vi "HW_Loop_20181101.vi"(7 "ErrorLocation":string="FPGA", 8 "error in (no error)":errorcluster, 9 "10MHzPLL?":bool, 10 "FPGA.Target":T1=enum."4", 11 "Queue in":refnum<queue>) -> (0 "error out":errorcluster)   [LabVIEW 2018]
uses:
  Queue/HWQueueElements.ctl
  Controls/Enums/TargetNumber.ctl
  Controls/HWCluster.ctl
  Controls/Clusts/FPGA_Config_Clust.ctl
  Queue/DataQueueElements.ctl
  Controls/Enums/NoiseQueueElements.ctl
  Controls/Clusts/Config_Clust.ctl
  Controls/Clusts/UserConfig.ctl
  Controls/PathsCluster.ctl
  Controls/Clusts/FrontPanel_UserConfig.ctl
  Controls/Clusts/Inclinometer_User_Cfg.ctl
  Controls/Clusts/FP_UserTargetConfig.ctl
  Controls/Clusts/FreqShift.ctl
  Controls/Clusts/FPGA_Scale.ctl
  Controls/Enums/ScaleMeasure.ctl
  Controls/RadioButtons/FilterEnableRadio.ctl
  Controls/Enums/WatchdogTimer_Enum.ctl
  <vilib>/FPGAPlugInAG/PXIe-7976R/niLvFpga_Open_PXIe-7976R.vi
  <vilib>/rvi/interface/common/dynamic/niFpgaDynamicAddResources.vi
  <vilib>/FPGAPlugInAG/Dynamic/niLvFpga_Reset_Dynamic.vi
  <vilib>/FPGAPlugInAG/Dynamic/niLvFpga_Run_Dynamic.vi
  <vilib>/FPGAPlugInAG/Dynamic/niLvFpga_Close_Dynamic.vi
  <vilib>/rvi/interface/nirviOpenFPGA/nirviOpenFPGA.xnode
  FPGA Bitfiles/20210518_00_ATA_FPGA.lvbitx
  <vilib>/rvi/interface/nirviMethod/nirviMethod.xnode
  <vilib>/rvi/interface/nirviCloseFPGA/nirviCloseFPGA.xnode
  <vilib>/rvi/interface/nirviReadWriteControl/nirviReadWriteControl.xnode
  NiFpgaLv.dll
  <vilib>/Utility/error.llb/Error Cluster From Error Code.vi
  <vilib>/rvi/interface/Simulation/niFpgaSimulationCallBeginRW.vi
  <vilib>/rvi/errors/niLvFpgaAdjustHostInterfaceError.vi
panel:
  out "Synthesizer Locked":bool
  out "HWLoopCount":i32
  out "# elements in queue":i32
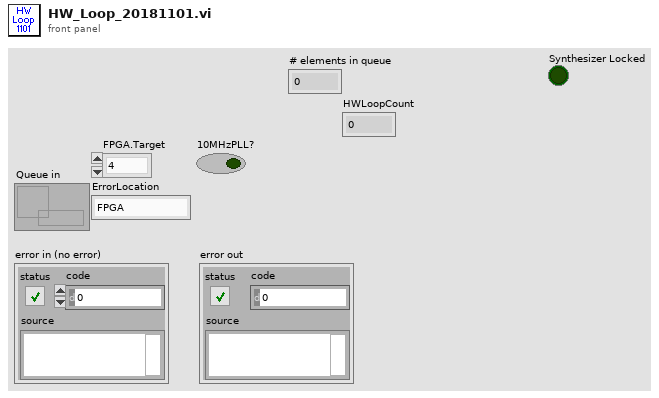
[diagram p1: front panel]
types:
  T1 = typedef "TargetNumber.ctl" = enum16{"1", "2", "3", "4"}
  T2 = typedef "HWCluster.ctl" = cluster{"FPGA":T3, "10MHzRef":bool, "FamInit":i32}
  T3 = typedef "FPGA_Config_Clust.ctl" = cluster{"Target":T1, "Channel":T1, "Ref1":refnum<k20>, "Ref2":refnum<k20>}
  T4 = typedef "HWQueueElements.ctl" = enum16{"HW_Init", "HW_UpdtCfg", "HW_Start", "HW_Pause", "HW_Run", "HW_Cls", "HW_Exit"}
  T5 = typedef "NoiseQueueElements.ctl" = enum16{"Noise_Startup", "Noise_Init", "Noise_Macro", "Noise_Config", "Noise_NewData", "Noise_Transform", "Noise_SumdTrace", "Noise_Send", "Noise_Probes", "Noise_Exit"}
  T6 = typedef "DataQueueElements.ctl" = enum16{"Data_Init", "Data_Config", "Data_AddData", "Data_FreqShift", "Data_FPGA_Write", "Data_Transform", "Data_Send", "Data_Exit"}
  T7 = enum8{"Internal Clock PLL Off", "Internal Clock PLL On (CLK_IN)", "External Clock (CLK_IN)", "Internal Clock PLL On (IoModSyncClk)"}
  T8 = typedef "Config_Clust.ctl" = cluster{"UsrCfg":T9, "FP_User":T11}
  T9 = typedef "UserConfig.ctl" = cluster{"Paths":T10, "SampleRate":dbl}
  T10 = typedef "PathsCluster.ctl" = cluster{"CfgFile":path, "LogFolder":path, "LogFile":path, "NAS path":path, "ThreshFile":path, "RedunFolder":path}
  T11 = typedef "FrontPanel_UserConfig.ctl" = cluster{"#NoiseSums":u32, "Max_df":u32, "AvgAvg":bool, "#Avg":u16, "AutoCenter":bool, "Inclin":T12, "1":T13, "2":T13, "3":T13, "4":T13, "Target to Probe":T1, "SNR_Thresh":dbl, "Paths":T10, "Connex_Location":string, "SimulateFPGA":bool, "Deadband":dbl}
  T12 = typedef "Inclinometer_User_Cfg.ctl" = cluster{"Vmin":dbl, "Vmax":dbl, "Angle_min":dbl, "Angle_max":dbl, "Offset":dbl, "Pos_Neg":bool}
  T13 = typedef "FP_UserTargetConfig.ctl" = cluster{"Cal_":T14, "Beac":T14, "Scale":T15, "Offset":fxp<+/-,16,16>, "Scale_Noise":fxp<+/-,30,30>, "Scale_Step1":fxp<+/-,17,17>, "Scale_In_RT":ext, "ScaleMeas":fxp<+/-,16,1>, "FreqsToRemove":i32[], "Width":i32[], "ScaleMeasEnum":T16, "FilterEnab":T17}
  T14 = typedef "FreqShift.ctl" = cluster{"Fine":dbl, "Coarse_":dbl}
  T15 = typedef "FPGA_Scale.ctl" = cluster{"Step4":fxp<+/-,23,23>, "Step5":fxp<+/-,23,23>, "Step6":fxp<+/-,23,23>, "Step7":fxp<+/-,23,23>}
  T16 = typedef "ScaleMeasure.ctl" = enum16{"1", "10", "50", "42"}
  T17 = typedef "FilterEnableRadio.ctl" = enum32{"None", "Step 1", "Frequency Shift", "Step 4", "Step 5", "Step 6", "Step 7"}
  T18 = typedef "WatchdogTimer_Enum.ctl" = enum16{"ResetAll", "CheckAll", "HW1", "HW2", "Tones", "FP", "Noise", "Log", "TCP", "AI", "TC", "ADAM", "Disdrom", "TE", "Weather"}
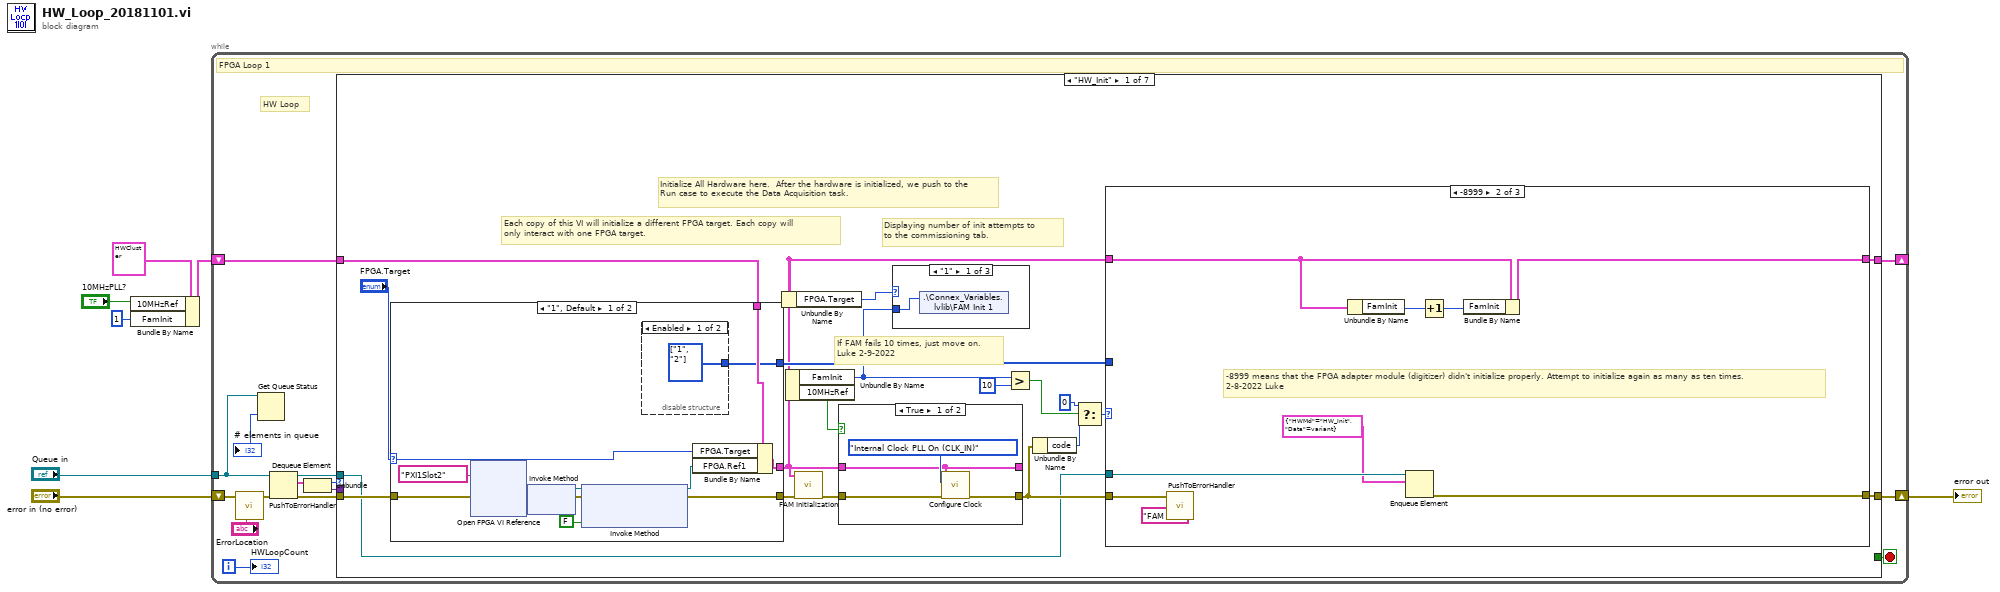
[diagram p0: block diagram]
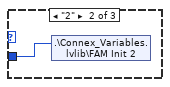
[diagram p2: hidden frame]
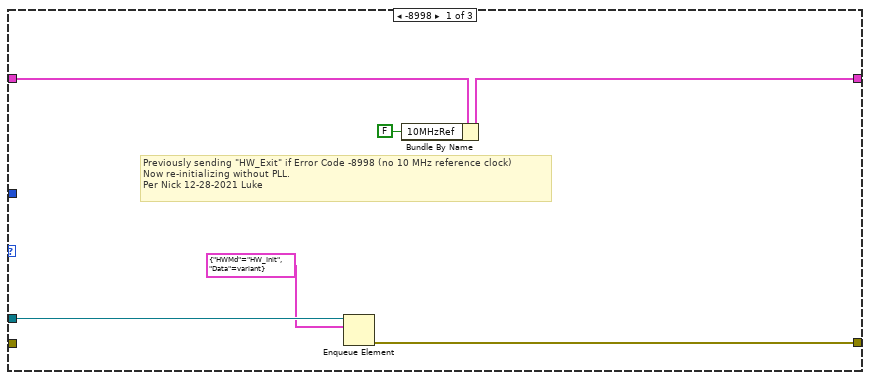
[diagram p4: hidden frame]
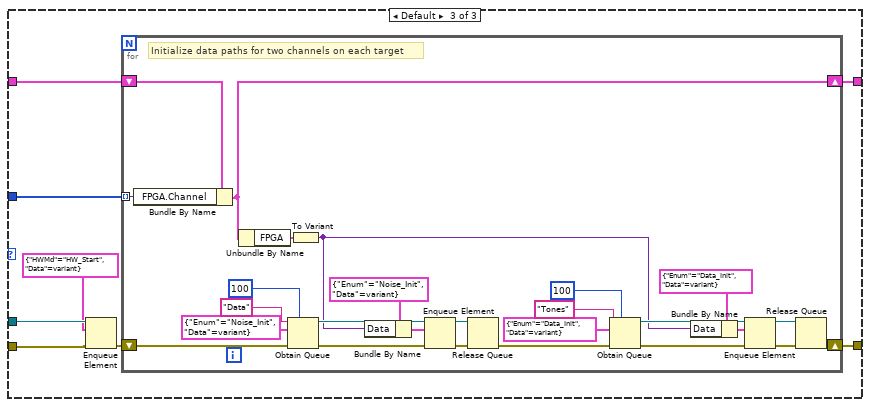
[diagram p5: hidden frame]
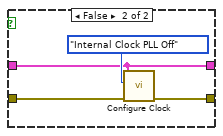
[diagram p6: hidden frame]
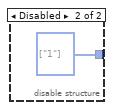
[diagram p7: hidden frame]
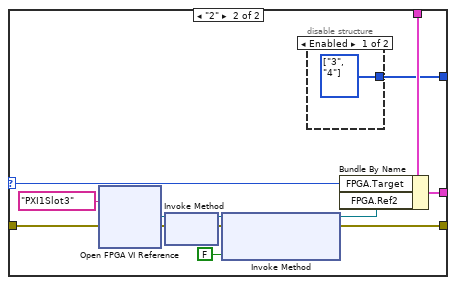
[diagram p8: hidden frame]
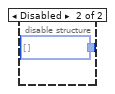
[diagram p9: hidden frame]
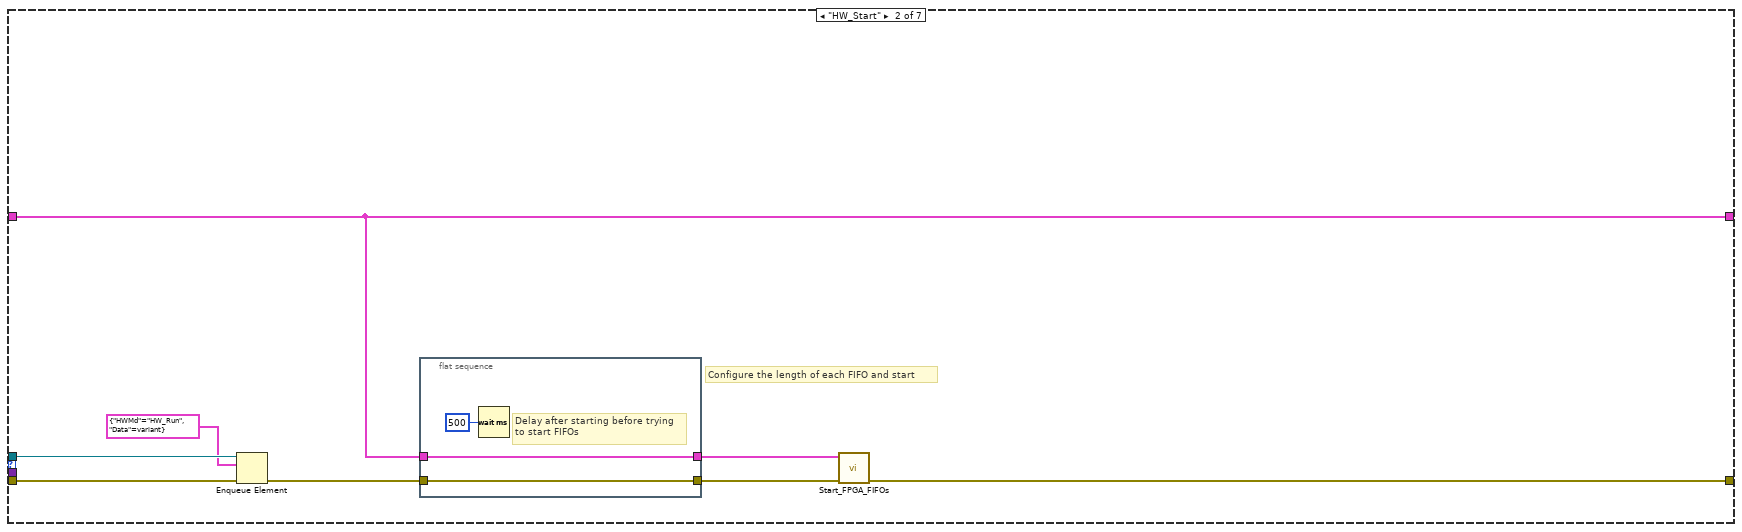
[diagram p10: hidden frame]
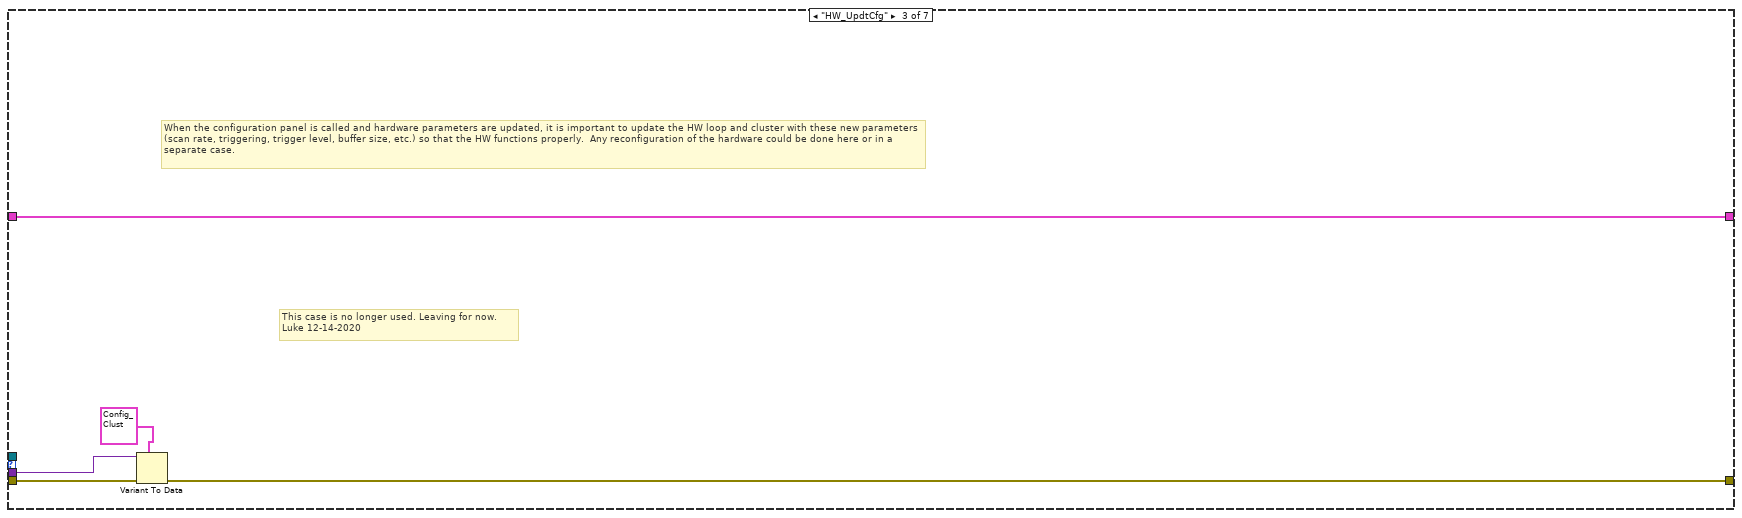
[diagram p11: hidden frame]
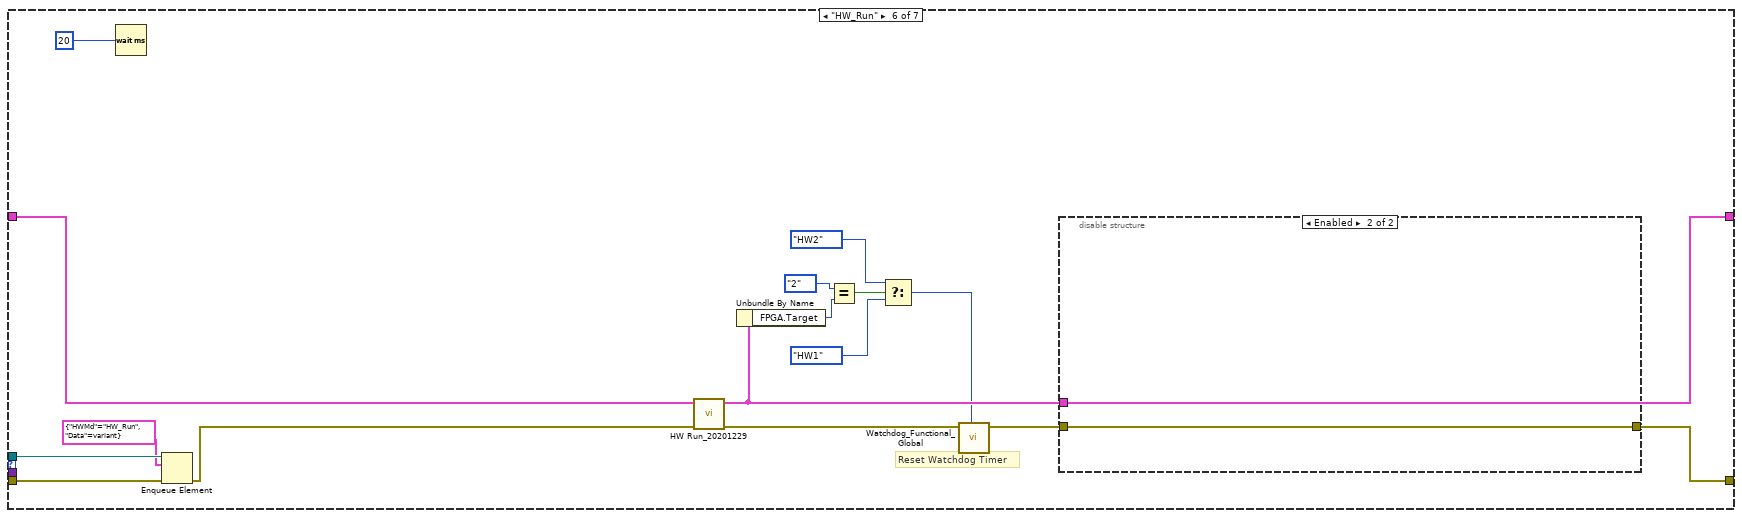
[diagram p14: hidden frame]
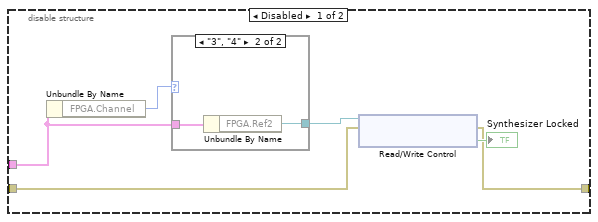
[diagram p15: hidden frame]
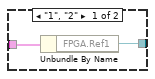
[diagram p16: hidden frame]
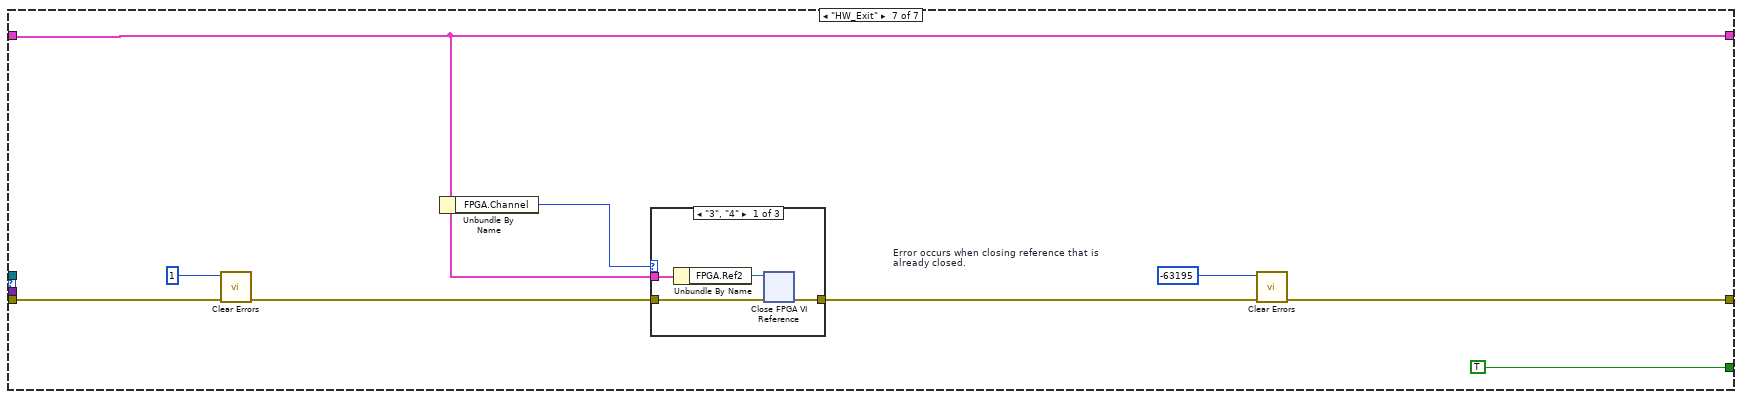
[diagram p17: hidden frame]
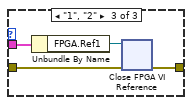
[diagram p19: hidden frame]
diagram:
  n1 = Bundle By Name(cluster=T2 {"FPGA"={"Target"=enum."4", "Channel"=enum."4", "Ref1"=refnum, "Ref2"=refnum}, "10MHzRef"=FALSE, "FamInit"=0} ("ClusterOut"), "10MHzRef"="10MHzPLL?", "FamInit"=1) -> (w3:T2)
  n2 = while {
    shift-right: [w12] -> w6
    shift-left: "error in (no error)" -> [w14]
    shift-right: [w22] -> _
    shift-left: w3 -> [w19]
    tunnel: "Queue in" -> [w10]
    i -> [w8]
    stop <- w15 stop-if-true
    # "HW Loop"
    # "FPGA Loop 1"
    n3 = call "PushToErrorHandler.vi"("ErrorIn"=w14, "ErrorLocation"="ErrorLocation") -> ("ErrorOut"=w13:errorcluster)  [unwired: 5 in]
    n4 = Get Queue Status(queue=w10) -> (# elements in queue=→"# elements in queue":i32)  [unwired: 2 in, 7 out]
    n5 = Dequeue Element(queue=w10, error in (no error)=w13) -> (queue out=w17:refnum<queue>, element=w21:cluster{"HWMd":T4, "Data":variant}, error out=w18:errorcluster)  [unwired: 2 out]
    n6 = Unbundle(w21) -> ("HWMd"=w20:T4, "Data"=w16:variant)
    n7 = case shown="\"HW_Init\"" w20 {
      tunnel: [w37 w138 w145 w148 w150 w160 w181] -> w12
      tunnel: [w36 w136 w142 w147 w149 w157 w179] -> w22
      tunnel: w19 -> [w39 w136 w142 w147 w149 w162 w179]
      tunnel: w18 -> [w41 w133 w146 w148 w150 w166 w178]
      tunnel: w17 -> [w31 w132 _ _ _ w165 _]
      tunnel: w16 -> [_ _ w144 _ _ _ _]
      tunnel: [_ _ _ _ _ _ TRUE ("Exit?")] -> w15
      frame "HW_Init" {
        # "Displaying number of init attempts to\nto the commissioning tab."
        # "If FAM fails 10 times, just move on.\nLuke 2-9-2022"
        # "Each copy of this VI will initialize a different FPGA target. Each copy will\nonly interact with one FPGA target."
        # "Initialize All Hardware here.  After the hardware is initialized, we push to the Run case to execute the Data Acquisition task."
        n8 = case shown="\"1\", Default" "FPGA.Target" {
          selector: "FPGA.Target" -> [w108 w123]
          tunnel: w41 -> [w113 w128]
          tunnel: [w103 w117] -> w38
          tunnel: w39 -> [w111 w127]
          tunnel: [w110 w126] -> w25
          tunnel: [w109 w124] -> w35
          frame "1", Default {
            n9 = xnode ("Open FPGA VI Reference")("error in"=w113, "resource name"=tag "PXI1Slot2") -> ("FPGA VI Reference Out"=w106:refnum<k20>, "error out"=w107:errorcluster)
            n10 = xnode "Invoke Method"("FPGA VI Reference In"=w106, "error in"=w107) -> ("FPGA VI Reference Out"=w104:refnum<k20>, "error out"=w105:errorcluster)
            n11 = xnode "Invoke Method"("FPGA VI Reference In"=w104, "error in"=w105, "Wait Until Done (F)"=FALSE) -> ("FPGA VI Reference Out"=w101:refnum<k20>, "error out"=w103:errorcluster)
            n12 = disable-structure shown="Enabled" {
              disable-tunnel: [w114 w115] -> w109
              frame Enabled {
                w114 = T1[] [enum."1", enum."2"] items=["1", "2", "3", "4"]
              }
              frame Disabled {
                w115 = T1[] [enum."1"] items=["1", "2", "3", "4"]
              }
            }
            n13 = Bundle By Name(cluster=w111, "FPGA.Target"=w108, "FPGA.Ref1"=w101) -> (w110:T2)
          }
          frame "2" {
            n14 = xnode ("Open FPGA VI Reference")("error in"=w128, "resource name"=tag "PXI1Slot3") -> ("FPGA VI Reference Out"=w121:refnum<k20>, "error out"=w122:errorcluster)
            n15 = xnode "Invoke Method"("FPGA VI Reference In"=w121, "error in"=w122) -> ("FPGA VI Reference Out"=w119:refnum<k20>, "error out"=w120:errorcluster)
            n16 = xnode "Invoke Method"("FPGA VI Reference In"=w119, "error in"=w120, "Wait Until Done (F)"=FALSE) -> ("FPGA VI Reference Out"=w118:refnum<k20>, "error out"=w117:errorcluster)
            n17 = disable-structure shown="Enabled" {
              disable-tunnel: [w129 w130] -> w124
              frame Enabled {
                w129 = T1[] [enum."3", enum."4"] items=["1", "2", "3", "4"]
              }
              frame Disabled {
                w130 = T1[] [] items=["1", "2", "3", "4"]
              }
            }
            n18 = Bundle By Name(cluster=w127, "FPGA.Target"=w123, "FPGA.Ref2"=w118) -> (w126:T2)
          }
        }
        n19 = Unbundle By Name(w25) -> ("FPGA.Target"=w24:T1)
        n20 = Unbundle By Name(w25) -> ("FamInit"=w23:i32, "10MHzRef"=w33:bool)
        n21 = call "FAM Initialization.vi"("error in (no error)"=w38, "Cluster"=w25) -> ("error out"=w34:errorcluster)  [unwired: 8 in, 1 out]
        n22 = case shown="True" w33 {
          tunnel: w34 -> [w94 w98]
          tunnel: [w95 w99] -> w32
          tunnel: w25 -> [w93 w97]
          tunnel: [w93 w97] -> _
          frame True {
            n23 = call "Configure Clock.vi"("error in"=w94, "Clock Source"=T7."Internal Clock PLL On (CLK_IN)", "Cluster"=w93) -> ("error out"=w95:errorcluster)  [unwired: 7 in, 1 out]
          }
          frame False {
            n24 = call "Configure Clock.vi"("error in"=w98, "Clock Source"=T7."Internal Clock PLL Off", "Cluster"=w97) -> ("error out"=w99:errorcluster)  [unwired: 7 in, 1 out]
          }
        }
        n25 = case shown="\"1\"" w24 {
          tunnel: w23 -> [w42 w43 _]
          frame "1" {
            n26 = shared-variable ".\\Connex_Variables.lvlib\\FAM Init 1"(w42) -> ()  [unwired: 1 in, 1 out]
          }
          frame "2" {
            n27 = shared-variable ".\\Connex_Variables.lvlib\\FAM Init 2"(w43) -> ()  [unwired: 1 in, 1 out]
          }
          frame Default {
          }
        }
        n28 = Greater?(x=w23, y=10) -> (0:w29:bool)
        n29 = Unbundle By Name(w32) -> ("code"=w28:i32)
        n30 = Select(t=0, s=w29, f=w28) -> (s? t:f=w27:i32)
        n31 = case shown="-8999" w27 {
          tunnel: [w48 w57 w66] -> w37
          tunnel: [w46 w56 w65] -> w36
          tunnel: w35 -> [_ _ w64]
          tunnel: w32 -> [_ w51 w61]
          tunnel: w25 -> [w47 w54 w63]
          tunnel: w31 -> [w49 w58 w60]
          frame -8998 {
            # "Previously sending \"HW_Exit\" if Error Code -8998 (no 10 MHz reference clock)\nNow re-initializing without PLL. \nPer Nick 12-28-2021 Luke"
            n32 = Enqueue Element(queue=w49, element=cluster{"HWMd":T4, "Data":variant} {"HWMd"=enum."HW_Init", "Data"=variant}) -> (error out=w48:errorcluster)  [unwired: 1 in, 3 out]
            n33 = Bundle By Name(cluster=w47, "10MHzRef"=FALSE) -> (w46:T2)
          }
          frame -8999 {
            # "-8999 means that the FPGA adapter module (digitizer) didn't initialize properly. Attempt to initialize again as many as ten times.\n2-8-2022 Luke"
            n34 = call "PushToErrorHandler.vi"("ErrorIn"=w51, "ErrorLocation"="FAM Init") -> ()  [unwired: 5 in, 1 out]
            n35 = Unbundle By Name(w54) -> ("FamInit"=w53:i32)
            n36 = Enqueue Element(queue=w58, element=cluster{"HWMd":T4, "Data":variant} {"HWMd"=enum."HW_Init", "Data"=variant}) -> (error out=w57:errorcluster)  [unwired: 1 in, 3 out]
            n37 = Increment(x=w53) -> (x+1=w52:i32)
            n38 = Bundle By Name(cluster=w54, "FamInit"=w52) -> (w56:T2)
          }
          frame Default {
            n39 = Enqueue Element(queue=w60, element=cluster{"HWMd":T4, "Data":variant} {"HWMd"=enum."HW_Start", "Data"=variant}, error in (no error)=w61) -> (error out=w62:errorcluster)  [unwired: 3 out]
            n40 = for {
              shift-right: [w71] -> w66
              shift-left: w62 -> [w76]
              shift-right: [w68] -> w65
              shift-left: w63 -> [w69]
              tunnel: w64 -> [w67] mode=indexing
              # "Initialize data paths for two channels on each target"
              n41 = Bundle By Name(cluster=w69, "FPGA.Channel"=w67) -> (w68:T2)
              n42 = Unbundle By Name(w68) -> ("FPGA"=w81:T3)
              n43 = Obtain Queue(max queue size (-1, unlimited)=100, name (unnamed)="Data", element data type=cluster{"Enum":T5, "Data":variant} {"Enum"=enum."Noise_Init", "Data"=variant}, error in (no error)=w76) -> (queue out=w80:refnum<queue>, error out=w82:errorcluster)  [unwired: 1 in, 1 out]
              n44 = To Variant(anything=w81) -> (Variant=w77:variant)
              n45 = Bundle By Name(cluster=cluster{"Enum":T5, "Data":variant} {"Enum"=enum."Noise_Init", "Data"=variant} ("element"), "Data"=w77) -> (w78:cluster{"Enum":T5, "Data":variant})
              n46 = Enqueue Element(queue=w80, element=w78, error in (no error)=w82) -> (queue out=w73:refnum<queue>, error out=w75:errorcluster)  [unwired: 2 out]
              n47 = Release Queue(queue=w73, error in (no error)=w75) -> (error out=w74:errorcluster)  [unwired: 1 in, 2 out]
              n48 = Obtain Queue(max queue size (-1, unlimited)=100, name (unnamed)="Tones", element data type=cluster{"Enum":T6, "Data":variant} {"Enum"=enum."Data_Init", "Data"=variant}, error in (no error)=w74) -> (queue out=w86:refnum<queue>, error out=w87:errorcluster)  [unwired: 1 in, 1 out]
              n49 = Bundle By Name(cluster=cluster{"Enum":T6, "Data":variant} {"Enum"=enum."Data_Init", "Data"=variant} ("element"), "Data"=w77) -> (w91:cluster{"Enum":T6, "Data":variant})
              n50 = Enqueue Element(queue=w86, element=w91, error in (no error)=w87) -> (queue out=w70:refnum<queue>, error out=w72:errorcluster)  [unwired: 2 out]
              n51 = Release Queue(queue=w70, error in (no error)=w72) -> (error out=w71:errorcluster)  [unwired: 1 in, 2 out]
            }
          }
        }
      }
      frame "HW_Start" {
        # "Configure the length of each FIFO and start"
        n52 = Enqueue Element(queue=w132, element=cluster{"HWMd":T4, "Data":variant} {"HWMd"=enum."HW_Run", "Data"=variant}, error in (no error)=w133) -> (error out=w134:errorcluster)  [unwired: 1 in, 2 out]
        n53 = flat-sequence {
          tunnel: w134 -> [w140]
          tunnel: [w140] -> w137
          tunnel: w136 -> [w139]
          tunnel: [w139] -> w135
          frame #0 {
            # "Delay after starting before trying\nto start FIFOs"
            n54 = Wait (ms)(milliseconds to wait=u32 500) -> ()  [unwired: 1 out]
          }
        }
        n55 = call "Start_FPGA_FIFOs.vi"("error in (no error)"=w137, "ClusterOut"=w135) -> ("error out"=w138:errorcluster)  [unwired: 9 in]
      }
      frame "HW_UpdtCfg" {
        # "This case is no longer used. Leaving for now.\nLuke 12-14-2020"
        # "When the configuration panel is called and hardware parameters are updated, it is important to update the HW loop and cluster with these new parameters (scan rate, triggering, trigger level, buffer size, etc.) so that the HW functions properly.  Any reconfiguration of the hardware could be done here or in a separate case."
        n56 = Variant To Data(error in=w146, type=T8 {"UsrCfg"={"Paths"={"CfgFile"=path "", "LogFolder"=path "", "LogFile"=path "", "NAS path"=path "", "ThreshFile"=path "", "RedunFolder"=path ""}, "SampleRate"=12500.0}, "FP_User"={"#NoiseSums"=1, "Max_df"=1, "AvgAvg"=FALSE, "#Avg"=1, "AutoCenter"=FALSE, "Inclin"={"Vmin"=0.0, "Vmax"=0.0, "Angle_min"=0.0, "Angle_max"=0.0, "Offset"=0.0, "Pos_Neg"=FALSE}, "1"={"Cal_"={"Fine"=0.000213623046875, "Coarse_"=4194303.0}, "Beac"={"Fine"=4194303.0, "Coarse_"=1.0}, "Scale"={"Step4"=10000.0, "Step5"=4194303.0, "Step6"=1.0, "Step7"=10000.0}, "Offset"=0.0, "Scale_Noise"=4194303.0, "Scale_Step1"=65535.0, "Scale_In_RT"=1.0, "ScaleMeas"=0.999969482421875, "FreqsToRemove"=[0, 1633], "Width"=[0, 1633], "ScaleMeasEnum"=enum."50", "FilterEnab"=enum."Step 1"}, "2"={"Cal_"={"Fine"=0.000213623046875, "Coarse_"=4194303.0}, "Beac"={"Fine"=0.000213623046875, "Coarse_"=4194303.0}, "Scale"={"Step4"=0.0, "Step5"=4194303.0, "Step6"=1.0, "Step7"=10000.0}, "Offset"=0.0, "Scale_Noise"=4194303.0, "Scale_Step1"=65535.0, "Scale_In_RT"=1.0, "ScaleMeas"=0.999969482421875, "FreqsToRemove"=[0, 1633], "Width"=[0, 1633], "ScaleMeasEnum"=enum."50", "FilterEnab"=enum."Step 1"}, "3"={"Cal_"={"Fine"=0.000213623046875, "Coarse_"=4194303.0}, "Beac"={"Fine"=0.000213623046875, "Coarse_"=4194303.0}, "Scale"={"Step4"=0.0, "Step5"=4194303.0, "Step6"=1.0, "Step7"=10000.0}, "Offset"=0.0, "Scale_Noise"=4194303.0, "Scale_Step1"=65535.0, "Scale_In_RT"=1.0, "ScaleMeas"=0.999969482421875, "FreqsToRemove"=[0, 1633], "Width"=[0, 1633], "ScaleMeasEnum"=enum."50", "FilterEnab"=enum."Step 1"}, "4"={"Cal_"={"Fine"=0.000213623046875, "Coarse_"=4194303.0}, "Beac"={"Fine"=0.000213623046875, "Coarse_"=4194303.0}, "Scale"={"Step4"=0.0, "Step5"=4194303.0, "Step6"=1.0, "Step7"=10000.0}, "Offset"=0.0, "Scale_Noise"=4194303.0, "Scale_Step1"=1.0, "Scale_In_RT"=10000.0, "ScaleMeas"=0.999969482421875, "FreqsToRemove"=[0, 1633], "Width"=[0, 1633], "ScaleMeasEnum"=enum."50", "FilterEnab"=enum."Step 1"}, "Target to Probe"=enum."4", "SNR_Thresh"=1.0, "Paths"={"CfgFile"=path "", "LogFolder"=path "", "LogFile"=path "", "NAS path"=path "", "ThreshFile"=path "", "RedunFolder"=path ""}, "Connex_Location"="", "SimulateFPGA"=FALSE, "Deadband"=0.0}} ("Config"), Variant=w144) -> (error out=w145:errorcluster)  [unwired: 1 out]
      }
      frame "HW_Cls" {
        # "Close All Hardware"
      }
      frame "HW_Pause" {
      }
      frame "HW_Run" {
        # "Reset Watchdog Timer"
        n57 = Wait (ms)(milliseconds to wait=u32 20) -> ()  [unwired: 1 out]
        n58 = Enqueue Element(queue=w165, element=cluster{"HWMd":T4, "Data":variant} {"HWMd"=enum."HW_Run", "Data"=variant}, error in (no error)=w166) -> (error out=w161:errorcluster)  [unwired: 3 out]
        n59 = call "HW Run_20201229.vi"("error in (no error)"=w161, "ClusterOut in"=w162) -> ("error out"=w159:errorcluster, "ClusterOut out"=w157:T2)  [unwired: 8 in]
        n60 = Unbundle By Name(w157) -> ("FPGA.Target"=w155:T1)
        n61 = Equal?(x=TargetNumber."2" ("FPGA.Target"), y=w155) -> (x = y?=w154:bool)
        n62 = Select(t=WatchdogTimer_Enum."HW2" ("Watchdog"), s=w154, f=WatchdogTimer_Enum."HW1" ("Watchdog")) -> (s? t:f=w151:T18)
        n63 = call "Watchdog_Functional_Global.vi"("Watchdog"=w151, "error in"=w159) -> ("error out"=w158:errorcluster)  [unwired: 7 in, 2 out]
        n64 = disable-structure shown="Enabled" {
          disable-tunnel: w157 -> [w171 _]
          disable-tunnel: w158 -> [w168 w177]
          disable-tunnel: [w167 w177] -> w160
          frame Disabled {
            n65 = Unbundle By Name(w171) -> ("FPGA.Channel"=w172:T1)
            n66 = case shown="\"3\", \"4\"" w172 {
              tunnel: w171 -> [w174 w176]
              tunnel: [w173 w175] -> w170
              frame "1", "2" {
                n67 = Unbundle By Name(w174) -> ("FPGA.Ref1"=w173:refnum<k20>)
              }
              frame "3", "4" {
                n68 = Unbundle By Name(w176) -> ("FPGA.Ref2"=w175:refnum<k20>)
              }
            }
            n69 = xnode "Read/Write Control"("FPGA VI Reference In"=w170, "error in"=w168) -> ("error out"=w167:errorcluster, "Synthesizer Locked"=→"Synthesizer Locked":bool)  [unwired: 1 out]
          }
          frame Enabled {
          }
        }
      }
      frame "HW_Exit" {
        w180 = -63195  # Error occurs when closing reference that is already closed.
        n70 = call <vilib>:"Clear Errors.vi"("error in (no error)"=w178, "specific error code to clear (0: all)"=1) -> ("error out"=w184:errorcluster)  [unwired: 4 in, 1 out]
        n71 = Unbundle By Name(w179) -> ("FPGA.Channel"=w182:T1)
        n72 = case shown="\"3\", \"4\"" w182 {
          tunnel: [w190 w191 w195] -> w185
          tunnel: w184 -> [w188 w191 w193]
          tunnel: w179 -> [w187 _ w192]
          frame "3", "4" {
            n73 = Unbundle By Name(w187) -> ("FPGA.Ref2"=w189:refnum<k20>)
            n74 = xnode ("Close FPGA VI Reference")("FPGA VI Reference In"=w189, "error in"=w188) -> ("error out"=w190:errorcluster)
          }
          frame Default {
            # "Don't try to close channel\nother than 1 & 2.\n(3&4 are redundant)"
          }
          frame "1", "2" {
            n75 = Unbundle By Name(w192) -> ("FPGA.Ref1"=w194:refnum<k20>)
            n76 = xnode ("Close FPGA VI Reference")("FPGA VI Reference In"=w194, "error in"=w193) -> ("error out"=w195:errorcluster)
          }
        }
        n77 = call <vilib>:"Clear Errors.vi"("error in (no error)"=w185, "specific error code to clear (0: all)"=w180) -> ("error out"=w181:errorcluster)  [unwired: 4 in, 1 out]
      }
    }
    "HWLoopCount" <- w8
  }
  "error out" <- w6
